vi "neuKLEIN.vi"() -> ()   [LabVIEW 2016] (continued)
"DIO2", "DIO3", "DIO4", "DIO5", "DIO6", "DIO7", "DIO8", "DIO9", "DIO10", "DIO11", "DIO12", "DIO13", "DIO14", "DIO15", "DIO16", "DIO17", "DIO18", "DIO19", "DIO20", "DIO21", "DIO22", "DIO23", "DIO24", "DIO25", "DIO26", "DIO27", "DIO28", "DIO29", "DIO30", "DIO31", "FALSE"]; "Channel 10"."Inputs" items=["DIO0", "DIO1", "DIO2", "DIO3", "DIO4", "DIO5", "DIO6", "DIO7", "DIO8", "DIO9", "DIO10", "DIO11", "DIO12", "DIO13", "DIO14", "DIO15", "DIO16", "DIO17", "DIO18", "DIO19", "DIO20", "DIO21", "DIO22", "DIO23", "DIO24", "DIO25", "DIO26", "DIO27", "DIO28", "DIO29", "DIO30", "DIO31", "FALSE"]; "Channel 10"."Operation" items=["OFF", "Constant", "Bool - Basic Switch", "Bool - AND Switch", "Bool - OR Switch", "Custom - Comp Basic Switch", "Custom - 461nm Freq."]; "Channel 9"."Input B" items=["DIO0", "DIO1", "DIO2", "DIO3", "DIO4", "DIO5", "DIO6", "DIO7", "DIO8", "DIO9", "DIO10", "DIO11", "DIO12", "DIO13", "DIO14", "DIO15", "DIO16", "DIO17", "DIO18", "DIO19", "DIO20", "DIO21", "DIO22", "DIO23", "DIO24", "DIO25", "DIO26", "DIO27", "DIO28", "DIO29", "DIO30", "DIO31", "FALSE"]; "Channel 9"."Input A" items=["DIO0", "DIO1", "DIO2", "DIO3", "DIO4", "DIO5", "DIO6", "DIO7", "DIO8", "DIO9", "DIO10", "DIO11", "DIO12", "DIO13", "DIO14", "DIO15", "DIO16", "DIO17", "DIO18", "DIO19", "DIO20", "DIO21", "DIO22", "DIO23", "DIO24", "DIO25", "DIO26", "DIO27", "DIO28", "DIO29", "DIO30", "DIO31", "FALSE"]; "Channel 9"."Inputs" items=["DIO0", "DIO1", "DIO2", "DIO3", "DIO4", "DIO5", "DIO6", "DIO7", "DIO8", "DIO9", "DIO10", "DIO11", "DIO12", "DIO13", "DIO14", "DIO15", "DIO16", "DIO17", "DIO18", "DIO19", "DIO20", "DIO21", "DIO22", "DIO23", "DIO24", "DIO25", "DIO26", "DIO27", "DIO28", "DIO29", "DIO30", "DIO31", "FALSE"]; "Channel 9"."Operation" items=["OFF", "Constant", "Bool - Basic Switch", "Bool - AND Switch", "Bool - OR Switch", "Custom - Comp Basic Switch", "Custom - 461nm Freq."]; "Channel 8"."Input B" items=["DIO0", "DIO1", "DIO2", "DIO3", "DIO4", "DIO5", "DIO6", "DIO7", "DIO8", "DIO9", "DIO10", "DIO11", "DIO12", "DIO13", "DIO14", "DIO15", "DIO16", "DIO17", "DIO18", "DIO19", "DIO20", "DIO21", "DIO22", "DIO23", "DIO24", "DIO25", "DIO26", "DIO27", "DIO28", "DIO29", "DIO30", "DIO31", "FALSE"]; "Channel 8"."Input A" items=["DIO0", "DIO1", "DIO2", "DIO3", "DIO4", "DIO5", "DIO6", "DIO7", "DIO8", "DIO9", "DIO10", "DIO11", "DIO12", "DIO13", "DIO14", "DIO15", "DIO16", "DIO17", "DIO18", "DIO19", "DIO20", "DIO21", "DIO22", "DIO23", "DIO24", "DIO25", "DIO26", "DIO27", "DIO28", "DIO29", "DIO30", "DIO31", "FALSE"]; "Channel 8"."Inputs" items=["DIO0", "DIO1", "DIO2", "DIO3", "DIO4", "DIO5", "DIO6", "DIO7", "DIO8", "DIO9", "DIO10", "DIO11", "DIO12", "DIO13", "DIO14", "DIO15", "DIO16", "DIO17", "DIO18", "DIO19", "DIO20", "DIO21", "DIO22", "DIO23", "DIO24", "DIO25", "DIO26", "DIO27", "DIO28", "DIO29", "DIO30", "DIO31", "FALSE"]; "Channel 8"."Operation" items=["OFF", "Constant", "Bool - Basic Switch", "Bool - AND Switch", "Bool - OR Switch", "Custom - Comp Basic Switch", "Custom - 461nm Freq."]; "Channel 7"."Input B" items=["DIO0", "DIO1", "DIO2", "DIO3", "DIO4", "DIO5", "DIO6", "DIO7", "DIO8", "DIO9", "DIO10", "DIO11", "DIO12", "DIO13", "DIO14", "DIO15", "DIO16", "DIO17", "DIO18", "DIO19", "DIO20", "DIO21", "DIO22", "DIO23", "DIO24", "DIO25", "DIO26", "DIO27", "DIO28", "DIO29", "DIO30", "DIO31", "FALSE"]; "Channel 7"."Input A" items=["DIO0", "DIO1", "DIO2", "DIO3", "DIO4", "DIO5", "DIO6", "DIO7", "DIO8", "DIO9", "DIO10", "DIO11", "DIO12", "DIO13", "DIO14", "DIO15", "DIO16", "DIO17", "DIO18", "DIO19", "DIO20", "DIO21", "DIO22", "DIO23", "DIO24", "DIO25", "DIO26", "DIO27", "DIO28", "DIO29", "DIO30", "DIO31", "FALSE"]; "Channel 7"."Inputs" items=["DIO0", "DIO1", "DIO2", "DIO3", "DIO4", "DIO5", "DIO6", "DIO7", "DIO8", "DIO9", "DIO10", "DIO11", "DIO12", "DIO13", "DIO14", "DIO15", "DIO16", "DIO17", "DIO18", "DIO19", "DIO20", "DIO21", "DIO22", "DIO23", "DIO24", "DIO25", "DIO26", "DIO27", "DIO28", "DIO29", "DIO30", "DIO31", "FALSE"]; "Channel 7"."Operation" items=["OFF", "Constant", "Bool - Basic Switch", "Bool - AND Switch", "Bool - OR Switch", "Custom - Comp Basic Switch", "Custom - 461nm Freq."]; "Channel 6"."Input B" items=["DIO0", "DIO1", "DIO2", "DIO3", "DIO4", "DIO5", "DIO6", "DIO7", "DIO8", "DIO9", "DIO10", "DIO11", "DIO12", "DIO13", "DIO14", "DIO15", "DIO16", "DIO17", "DIO18", "DIO19", "DIO20", "DIO21", "DIO22", "DIO23", "DIO24", "DIO25", "DIO26", "DIO27", "DIO28", "DIO29", "DIO30", "DIO31", "FALSE"]; "Channel 6"."Input A" items=["DIO0", "DIO1", "DIO2", "DIO3", "DIO4", "DIO5", "DIO6", "DIO7", "DIO8", "DIO9", "DIO10", "DIO11", "DIO12", "DIO13", "DIO14", "DIO15", "DIO16", "DIO17", "DIO18", "DIO19", "DIO20", "DIO21", "DIO22", "DIO23", "DIO24", "DIO25", "DIO26", "DIO27", "DIO28", "DIO29", "DIO30", "DIO31", "FALSE"]; "Channel 6"."Inputs" items=["DIO0", "DIO1", "DIO2", "DIO3", "DIO4", "DIO5", "DIO6", "DIO7", "DIO8", "DIO9", "DIO10", "DIO11", "DIO12", "DIO13", "DIO14", "DIO15", "DIO16", "DIO17", "DIO18", "DIO19", "DIO20", "DIO21", "DIO22", "DIO23", "DIO24", "DIO25", "DIO26", "DIO27", "DIO28", "DIO29", "DIO30", "DIO31", "FALSE"]; "Channel 6"."Operation" items=["OFF", "Constant", "Bool - Basic Switch", "Bool - AND Switch", "Bool - OR Switch", "Custom - Comp Basic Switch", "Custom - 461nm Freq."]; "Channel 5"."Input B" items=["DIO0", "DIO1", "DIO2", "DIO3", "DIO4", "DIO5", "DIO6", "DIO7", "DIO8", "DIO9", "DIO10", "DIO11", "DIO12", "DIO13", "DIO14", "DIO15", "DIO16", "DIO17", "DIO18", "DIO19", "DIO20", "DIO21", "DIO22", "DIO23", "DIO24", "DIO25", "DIO26", "DIO27", "DIO28", "DIO29", "DIO30", "DIO31", "FALSE"]; "Channel 5"."Input A" items=["DIO0", "DIO1", "DIO2", "DIO3", "DIO4", "DIO5", "DIO6", "DIO7", "DIO8", "DIO9", "DIO10", "DIO11", "DIO12", "DIO13", "DIO14", "DIO15", "DIO16", "DIO17", "DIO18", "DIO19", "DIO20", "DIO21", "DIO22", "DIO23", "DIO24", "DIO25", "DIO26", "DIO27", "DIO28", "DIO29", "DIO30", "DIO31", "FALSE"]; "Channel 5"."Inputs" items=["DIO0", "DIO1", "DIO2", "DIO3", "DIO4", "DIO5", "DIO6", "DIO7", "DIO8", "DIO9", "DIO10", "DIO11", "DIO12", "DIO13", "DIO14", "DIO15", "DIO16", "DIO17", "DIO18", "DIO19", "DIO20", "DIO21", "DIO22", "DIO23", "DIO24", "DIO25", "DIO26", "DIO27", "DIO28", "DIO29", "DIO30", "DIO31", "FALSE"]; "Channel 5"."Operation" items=["OFF", "Constant", "Bool - Basic Switch", "Bool - AND Switch", "Bool - OR Switch", "Custom - Comp Basic Switch", "Custom - 461nm Freq."]; "Channel 4"."Input B" items=["DIO0", "DIO1", "DIO2", "DIO3", "DIO4", "DIO5", "DIO6", "DIO7", "DIO8", "DIO9", "DIO10", "DIO11", "DIO12", "DIO13", "DIO14", "DIO15", "DIO16", "DIO17", "DIO18", "DIO19", "DIO20", "DIO21", "DIO22", "DIO23", "DIO24", "DIO25", "DIO26", "DIO27", "DIO28", "DIO29", "DIO30", "DIO31", "FALSE"]; "Channel 4"."Input A" items=["DIO0", "DIO1", "DIO2", "DIO3", "DIO4", "DIO5", "DIO6", "DIO7", "DIO8", "DIO9", "DIO10", "DIO11", "DIO12", "DIO13", "DIO14", "DIO15", "DIO16", "DIO17", "DIO18", "DIO19", "DIO20", "DIO21", "DIO22", "DIO23", "DIO24", "DIO25", "DIO26", "DIO27", "DIO28", "DIO29", "DIO30", "DIO31", "FALSE"]; "Channel 4"."Inputs" items=["DIO0", "DIO1", "DIO2", "DIO3", "DIO4", "DIO5", "DIO6", "DIO7", "DIO8", "DIO9", "DIO10", "DIO11", "DIO12", "DIO13", "DIO14", "DIO15", "DIO16", "DIO17", "DIO18", "DIO19", "DIO20", "DIO21", "DIO22", "DIO23", "DIO24", "DIO25", "DIO26", "DIO27", "DIO28", "DIO29", "DIO30", "DIO31", "FALSE"]; "Channel 4"."Operation" items=["OFF", "Constant", "Bool - Basic Switch", "Bool - AND Switch", "Bool - OR Switch", "Custom - Comp Basic Switch", "Custom - 461nm Freq."]; "Channel 3"."Input B" items=["DIO0", "DIO1", "DIO2", "DIO3", "DIO4", "DIO5", "DIO6", "DIO7", "DIO8", "DIO9", "DIO10", "DIO11", "DIO12", "DIO13", "DIO14", "DIO15", "DIO16", "DIO17", "DIO18", "DIO19", "DIO20", "DIO21", "DIO22", "DIO23", "DIO24", "DIO25", "DIO26", "DIO27", "DIO28", "DIO29", "DIO30", "DIO31", "FALSE"]; "Channel 3"."Input A" items=["DIO0", "DIO1", "DIO2", "DIO3", "DIO4", "DIO5", "DIO6", "DIO7", "DIO8", "DIO9", "DIO10", "DIO11", "DIO12", "DIO13", "DIO14", "DIO15", "DIO16", "DIO17", "DIO18", "DIO19", "DIO20", "DIO21", "DIO22", "DIO23", "DIO24", "DIO25", "DIO26", "DIO27", "DIO28", "DIO29", "DIO30", "DIO31", "FALSE"]; "Channel 3"."Inputs" items=["DIO0", "DIO1", "DIO2", "DIO3", "DIO4", "DIO5", "DIO6", "DIO7", "DIO8", "DIO9", "DIO10", "DIO11", "DIO12", "DIO13", "DIO14", "DIO15", "DIO16", "DIO17", "DIO18", "DIO19", "DIO20", "DIO21", "DIO22", "DIO23", "DIO24", "DIO25", "DIO26", "DIO27", "DIO28", "DIO29", "DIO30", "DIO31", "FALSE"]; "Channel 3"."Operation" items=["OFF", "Constant", "Bool - Basic Switch", "Bool - AND Switch", "Bool - OR Switch", "Custom - Comp Basic Switch", "Custom - 461nm Freq."]; "Channel 2"."Input B" items=["DIO0", "DIO1", "DIO2", "DIO3", "DIO4", "DIO5", "DIO6", "DIO7", "DIO8", "DIO9", "DIO10", "DIO11", "DIO12", "DIO13", "DIO14", "DIO15", "DIO16", "DIO17", "DIO18", "DIO19", "DIO20", "DIO21", "DIO22", "DIO23", "DIO24", "DIO25", "DIO26", "DIO27", "DIO28", "DIO29", "DIO30", "DIO31", "FALSE"]; "Channel 2"."Input A" items=["DIO0", "DIO1", "DIO2", "DIO3", "DIO4", "DIO5", "DIO6", "DIO7", "DIO8", "DIO9", "DIO10", "DIO11", "DIO12", "DIO13", "DIO14", "DIO15", "DIO16", "DIO17", "DIO18", "DIO19", "DIO20", "DIO21", "DIO22", "DIO23", "DIO24", "DIO25", "DIO26", "DIO27", "DIO28", "DIO29", "DIO30", "DIO31", "FALSE"]; "Channel 2"."Inputs" items=["DIO0", "DIO1", "DIO2", "DIO3", "DIO4", "DIO5", "DIO6", "DIO7", "DIO8", "DIO9", "DIO10", "DIO11", "DIO12", "DIO13", "DIO14", "DIO15", "DIO16", "DIO17", "DIO18", "DIO19", "DIO20", "DIO21", "DIO22", "DIO23", "DIO24", "DIO25", "DIO26", "DIO27", "DIO28", "DIO29", "DIO30", "DIO31", "FALSE"]; "Channel 2"."Operation" items=["OFF", "Constant", "Bool - Basic Switch", "Bool - AND Switch", "Bool - OR Switch", "Custom - Comp Basic Switch", "Custom - 461nm Freq."]; "Channel 1"."Input B" items=["DIO0", "DIO1", "DIO2", "DIO3", "DIO4", "DIO5", "DIO6", "DIO7", "DIO8", "DIO9", "DIO10", "DIO11", "DIO12", "DIO13", "DIO14", "DIO15", "DIO16", "DIO17", "DIO18", "DIO19", "DIO20", "DIO21", "DIO22", "DIO23", "DIO24", "DIO25", "DIO26", "DIO27", "DIO28", "DIO29", "DIO30", "DIO31", "FALSE"]; "Channel 1"."Input A" items=["DIO0", "DIO1", "DIO2", "DIO3", "DIO4", "DIO5", "DIO6", "DIO7", "DIO8", "DIO9", "DIO10", "DIO11", "DIO12", "DIO13", "DIO14", "DIO15", "DIO16", "DIO17", "DIO18", "DIO19", "DIO20", "DIO21", "DIO22", "DIO23", "DIO24", "DIO25", "DIO26", "DIO27", "DIO28", "DIO29", "DIO30", "DIO31", "FALSE"]; "Channel 1"."Inputs" items=["DIO0", "DIO1", "DIO2", "DIO3", "DIO4", "DIO5", "DIO6", "DIO7", "DIO8", "DIO9", "DIO10", "DIO11", "DIO12", "DIO13", "DIO14", "DIO15", "DIO16", "DIO17", "DIO18", "DIO19", "DIO20", "DIO21", "DIO22", "DIO23", "DIO24", "DIO25", "DIO26", "DIO27", "DIO28", "DIO29", "DIO30", "DIO31", "FALSE"]; "Channel 1"."Operation" items=["OFF", "Constant", "Bool - Basic Switch", "Bool - AND Switch", "Bool - OR Switch", "Custom - Comp Basic Switch", "Custom - 461nm Freq."]; "Channel 0"."Input B" items=["DIO0", "DIO1", "DIO2", "DIO3", "DIO4", "DIO5", "DIO6", "DIO7", "DIO8", "DIO9", "DIO10", "DIO11", "DIO12", "DIO13", "DIO14", "DIO15", "DIO16", "DIO17", "DIO18", "DIO19", "DIO20", "DIO21", "DIO22", "DIO23", "DIO24", "DIO25", "DIO26", "DIO27", "DIO28", "DIO29", "DIO30", "DIO31", "FALSE"]; "Channel 0"."Input A" items=["DIO0", "DIO1", "DIO2", "DIO3", "DIO4", "DIO5", "DIO6", "DIO7", "DIO8", "DIO9", "DIO10", "DIO11", "DIO12", "DIO13", "DIO14", "DIO15", "DIO16", "DIO17", "DIO18", "DIO19", "DIO20", "DIO21", "DIO22", "DIO23", "DIO24", "DIO25", "DIO26", "DIO27", "DIO28", "DIO29", "DIO30", "DIO31", "FALSE"]; "Channel 0"."Inputs" items=["DIO0", "DIO1", "DIO2", "DIO3", "DIO4", "DIO5", "DIO6", "DIO7", "DIO8", "DIO9", "DIO10", "DIO11", "DIO12", "DIO13", "DIO14", "DIO15", "DIO16", "DIO17", "DIO18", "DIO19", "DIO20", "DIO21", "DIO22", "DIO23", "DIO24", "DIO25", "DIO26", "DIO27", "DIO28", "DIO29", "DIO30", "DIO31", "FALSE"]; "Channel 0"."Operation" items=["OFF", "Constant", "Bool - Basic Switch", "Bool - AND Switch", "Bool - OR Switch", "Custom - Comp Basic Switch", "Custom - 461nm Freq."]}
  in  "FPGA_Labels":T34={"Channel 0"={"Channel Description"="This channel is outputtnig a constant voltage for unknown reasons\n- Jim\n2018.04.24"}, "Channel 1"={"Channel Description"="This channel is outputtnig a constant voltage for unknown reasons\n- Jim\n2018.04.24"}, "Channel 2"={"Channel Description"="Blue MOT Field Gradient"}, "Channel 3"={"Channel Description"="6221 Waveform trigger\n\nODT card that is triggered if either the sheet or the loading trap is turned on"}, "Channel 4"={"Channel Description"="X Trim Coil\nUsing Bio chip supply\n\n2018.04.12 - Zero field value\n-0.109985 V\n"}, "Channel 6"={"Channel Description"="Z Trim Coil\nUsing Gwinstek 5A supply\n\n2018.04.12 - Zero field value\n1.21 V\n\nODT loading value - 1.175 V\n2018.07.12 - Trapping 87\nTrap final: 81.8 MHz\nStir final:  143.605 MHz"}, "Channel 5"={"Channel Description"="Y Trim Coil\nUsing Gwinstek 3A supply\n\n2018.04.12 - Zero field value\n1.5 V\n"}, "Channel 7"={"Channel Description"="LCR Control\n\nDefining a coord systme with +Bz anti-parallel to gravity then\n\nSigma Plus:      1.75V\nSigma Minus:   0.95V"}, "Channel 8"={"Channel Description"="Blue Laser Frequency Selector\n\nSingle isotope without Cold MOT frequency shift can use the Bool - Basic switch operation\n\nDual isotopr or use of the Cold MOT freq shift should use the Custom 461nm Freq operation\n\nBool - Basic Switch op Outputs\nHI - Trap Freq.\nLO - Image Freq.\n\nCustom op Outputs:\n0 - Image Freq. 0\n1 - Image Freq. 1\n2 - Cold MOT Trap Freq\n3 - Hot MOT Trap Freq 0\n4 - Hot MOT Trap Freq 1\n"}, "Channel 9"={"Channel Description"="Blue MOT Power Control"}, "Channel 10"={"Channel Description"=""}, "Channel 11"={"Channel Description"=""}, "Channel 12"={"Channel Description"=""}, "Channel 13"={"Channel Description"=""}, "Channel 14"={"Channel Description"=""}, "Channel 15"={"Channel Description"=""}}
  in  "Synth Notes":string="- When scanning\nPhase to Change picks which synth to vary\nChannel to change picks the synth channel\n--------------------------------------------------------------------------\nNOTE: Signs below indicate the orientation of the AOM\n689 Master is locked -82 MHz of the 88Sr transition\n--------------------------------------------------------------------------\n## Constant values (i.e. important and generally unchanging)\n## Old sat abs parameters\n- Red Sat Abs. Freqs, Chan0: -81.85 MHz, Chan1: -82.15 MHz\n\n## New sat abs synth params as of 2018.08.22\n- Red Sat Abs. Chan0: 81.5MHz 1Vpp, Chan1: 82.5MHz 0.75Vpp\n\n- Isotope Selector AOM Freqs (2017.10.02)\n(note this value is sent through a doubler before gonig to the AOM)\n84Sr:  -93.745 MHz (\n86Sr:  no shift\n88Sr:  +82 MHz\n\n- Red MOT Single Freq. Resonances (2018.05.14)\nBoson: -82 MHz\nTrap: +82 MHz\nStir: +143.71 MHz\n\n- Slave 1 Inj. Freq  (2018.07.12),  +160 MHz \n\n--------------------------------------------------------------------------\n## Experimental Setting notes\n"
  in  "Novatech Synth Settings":T36[][](array[typedef])=[[{"Channel Settings"=[{"Voltage (Amp.) "=0.1, "Frequency (MHz)"=143.6, "Phase (deg)"=0.0, "Nickname"="SpinPol HI-Pump"}, {"Voltage (Amp.) "=1.0, "Frequency (MHz)"=0.0, "Phase (deg)"=0.0, "Nickname"="reserved for TM"}, {"Voltage (Amp.) "=0.1, "Frequency (MHz)"=145.0, "Phase (deg)"=0.0, "Nickname"="SpinPol LO-Probe"}, {"Voltage (Amp.) "=1.0, "Frequency (MHz)"=40.0, "Phase (deg)"=0.0, "Nickname"="Spec Offset Freq."}], "Active Chans"=[FALSE, FALSE, FALSE, TRUE], "COM Port"="ntSynth_COM5", "Table Mode"={"Initial Freq.(MHz)"=142.4, "FinalFreq"=145.32, "Freq. Step (MHz)"=0.365, "Voltage (Amp.)"=0.1, "Asc. & Desc."=FALSE, "Custom Frequencies"=[], "Custom Amplitude"=[], "Table Mode Switch"=FALSE, "Array Gen"=enum."Auto", "Randomize"=FALSE, "Continuous"=FALSE}}, {"Channel Settings"=[{"Voltage (Amp.) "=1.0, "Frequency (MHz)"=81.5, "Phase (deg)"=0.0, "Nickname"="Red Sat Abs - Chan0"}, {"Voltage (Amp.) "=0.97, "Frequency (MHz)"=82.5, "Phase (deg)"=0.0, "Nickname"="Red Sat Abs - Chan1"}, {"Voltage (Amp.) "=0.0, "Frequency (MHz)"=93.745, "Phase (deg)"=0.0, "Nickname"="Isotope Sel. AOM"}, {"Voltage (Amp.) "=0.28, "Frequency (MHz)"=160.0, "Phase (deg)"=0.0, "Nickname"="Slave 1 Inj. Freq"}], "Active Chans"=[FALSE, FALSE, FALSE, FALSE], "COM Port"="ntSynth_COM6", "Table Mode"={"Initial Freq.(MHz)"=0.0, "FinalFreq"=0.0, "Freq. Step (MHz)"=0.0, "Voltage (Amp.)"=0.0, "Asc. & Desc."=FALSE, "Custom Frequencies"=[], "Custom Amplitude"=[], "Table Mode Switch"=FALSE, "Array Gen"=enum."Auto", "Randomize"=FALSE, "Continuous"=FALSE}}], [{"Channel Settings"=[{"Voltage (Amp.) "=1.0, "Frequency (MHz)"=82.015, "Phase (deg)"=0.0, "Nickname"="Red Boson SF"}, {"Voltage (Amp.) "=1.0, "Frequency (MHz)"=100.0, "Phase (deg)"=0.0, "Nickname"="BROKEN"}, {"Voltage (Amp.) "=1.0, "Frequency (MHz)"=81.93, "Phase (deg)"=0.0, "Nickname"="Red 87 SF Trap"}, {"Voltage (Amp.) "=1.0, "Frequency (MHz)"=143.715, "Phase (deg)"=0.0, "Nickname"="Red 87 SF Stir"}], "Active Chans"=[TRUE, FALSE, TRUE, TRUE], "COM Port"="ntSynth_COM11", "Table Mode"={"Initial Freq.(MHz)"=0.17, "FinalFreq"=81.95, "Freq. Step (MHz)"=0.175, "Voltage (Amp.)"=0.0, "Asc. & Desc."=FALSE, "Custom Frequencies"=[], "Custom Amplitude"=[], "Table Mode Switch"=FALSE, "Array Gen"=enum."Auto", "Randomize"=FALSE, "Continuous"=FALSE}}, {"Channel Settings"=[{"Voltage (Amp.) "=0.22, "Frequency (MHz)"=85.95, "Phase (deg)"=0.0, "Nickname"="Spec. 1 Freq 0 (LO)"}, {"Voltage (Amp.) "=0.22, "Frequency (MHz)"=85.85, "Phase (deg)"=0.0, "Nickname"="Spec. 1 Freq 1 (HI)"}, {"Voltage (Amp.) "=1.0, "Frequency (MHz)"=93.745, "Phase (deg)"=0.0, "Nickname"="Bragg - 1"}, {"Voltage (Amp.) "=1.0, "Frequency (MHz)"=90.0, "Phase (deg)"=0.0, "Nickname"="Bragg - 2"}], "Active Chans"=[TRUE, TRUE, FALSE, FALSE], "COM Port"="ntSynth_COM10", "Table Mode"={"Initial Freq.(MHz)"=81.95, "FinalFreq"=82.05, "Freq. Step (MHz)"=0.002, "Voltage (Amp.)"=1.0, "Asc. & Desc."=TRUE, "Custom Frequencies"=[], "Custom Amplitude"=[], "Table Mode Switch"=FALSE, "Array Gen"=enum."Auto", "Randomize"=FALSE, "Continuous"=TRUE}}]] {"Table Mode"."Freq. Step (MHz)" format="%#_9g"; "Table Mode"."FinalFreq" format="%#_9g"; "Table Mode"."Initial Freq.(MHz)" format="%#_9g"; "Channel Settings"."Frequency (MHz)" format="%#_9g"}
  in  "Intitialize PicoScope":bool
  in  "PicoScope":T39={"Channel A Settings"={"Enabled"=FALSE, "Coupling"=1, "Range"=6, "Analogue Offset"=0.0}, "Channel B Settings"={"Enabled"=TRUE, "Coupling"=1, "Range"=8, "Analogue Offset"=0.0}, "Trigger Options"={"Trigger Enabled"=TRUE, "Trigger Source"=enum."Ext.", "Trigger Threshold (-5 to 5 V)"=1.0, "Trigger Slope"=2, "Trigger Delay (s)"=0.0, "Auto Trigger Time (ms)"=5000}, "Pico Scope Inititalization Settings"={"USB Power"=TRUE, "Use Serial Number"=FALSE, "Resolution"=3, "Serial Number"="", "Handle"=16384}, "Use PicoScope?"=FALSE, "Acquisition Settings"={"Pre Trigger Time (s)"=0.0, "Post Trigger Time (s)"=0.2, "Resolution (s)"=1e-06, "Four Channel Device"=FALSE, "Number of Captures"=1.0}} {"Acquisition Settings"."Number of Captures" min=1.0 step=1.0; "Acquisition Settings"."Resolution (s)" min=8e-09 max=34.36 step=8e-09 format="%#_6p"; "Acquisition Settings"."Post Trigger Time (s)" min=0.0 format="%#_6p"; "Acquisition Settings"."Pre Trigger Time (s)" min=0.0 format="%#_6p"; "Pico Scope Inititalization Settings"."Resolution" items=["8-bit", "12-bit", "14-bit", "15-bit (max. 2 ch.)", "16-bit (max. 1 ch.)"]; "Trigger Options"."Trigger Delay (s)" format="%.0p"; "Trigger Options"."Trigger Slope" items=["Rising"=2, "Falling"=3]; "Trigger Options"."Trigger Threshold (-5 to 5 V)" format="%.2f"; "Channel B Settings"."Range" items=["10 mV", "20 mV", "50 mV", "100 mV", "200 mV", "500 mV", "1 V", "2 V", "5 V", "10 V", "20 V", "50 V ", "100 V"]; "Channel B Settings"."Coupling" items=["AC", "DC"]; "Channel A Settings"."Range" items=["10 mV", "20 mV", "50 mV", "100 mV", "200 mV", "500 mV", "1 V", "2 V", "5 V", "10 V", "20 V", "50 V ", "100 V"]; "Channel A Settings"."Coupling" items=["AC", "DC"]}
  in  "Program Agilent":bool
  in  "Agilent E3631A Settings":T43={"VISA resource name"="Agilent_Trim_Supply", "Voltage Set (6V max)"=6.0, "Current Set (5A max)"=0.013, "Voltage Set (25V max)"=25.0, "Current Set (1A max)"=0.273, "Voltage Set (-25V max)"=-25.0, "Current Set (1A max)"=0.555, "6V Switch"=TRUE, "+25V Switch"=TRUE, "-25V Switch"=FALSE, "Agilent E3631A Measurements"={"6V Actual Voltage Level (V)"=0.02291032, "6V Actual Current Level (A)"=0.01098386, "25V Actual Voltage Level (V)"=0.4245154, "25V Actual Current Level (A)"=0.2743926, "-25V Actual Current Level (A)"=0.0, "-25V Actual Voltage Level (V)"=0.0}, "Triggered Agilent Settings"={"Trigger \nDelay (s)"=3.0, "Enable +6V Channel"=TRUE, "+6V Current"=0.02, "Enable -25V Channel"=TRUE, "-25V Current"=0.0, "Enable +25V Channel"=TRUE, "+25V Current"=0.275}, "Auto Program Agilent"=FALSE, "Agilent Software Trigger"=FALSE} {"Triggered Agilent Settings"."Trigger \nDelay (s)" min=0.0 max=3600.0 step=1.0 format="%.2f"; "Agilent E3631A Measurements"."-25V Actual Current Level (A)" format="%.3g"; "Agilent E3631A Measurements"."-25V Actual Voltage Level (V)" format="%.3g"; "Agilent E3631A Measurements"."25V Actual Current Level (A)" format="%.3g"; "Agilent E3631A Measurements"."25V Actual Voltage Level (V)" format="%.3g"; "Agilent E3631A Measurements"."6V Actual Current Level (A)" format="%.3g"; "Agilent E3631A Measurements"."6V Actual Voltage Level (V)" format="%.3g"; "Current Set (1A max)" format="%.3g"; "Voltage Set (-25V max)" format="%.3g"; "Current Set (1A max)" format="%.3g"; "Voltage Set (25V max)" format="%.3g"; "Current Set (5A max)" format="%.3g"; "Voltage Set (6V max)" format="%.3g"}
  in  "SaveButton":bool
  in  "XML Filename":string="20181207 - Settings 2"
  in  "Load":bool
  in  "XML File Location":path=path "Z:/Neutral/Experiment_Data/NeuKLEIN XML Configs/20181206 - test3 - SpinalCol MD5 0d3911740401e8bd5a903395efd23ac1.dat"
  out "current spinal_column MD5":string="0d3911740401e8bd5a903395efd23ac1"
  out "cRIO Ready":bool
  out "Picoscope Ready":bool
  in  "Break Loop":bool
  in  "Abort Scan":bool
  in  "Take Pictures":bool=TRUE
  in  "Trigger Snap Mode":bool=TRUE
  in  "Shutdown Experiment":bool
  in  "Start Experiment":bool
  out "Camera Ready":bool=TRUE
  out "Exp Running":bool
  in  "output cluster":T46
  in  "Stats Flag":bool
  out "Num and Temp Stats":T47 {"Std. Y Temp" format="%#_3p"; "Mean Y Temp" format="%#_3p"; "Mean X Temp" format="%#_3p"; "Mean Num." format="%^#.3e"; "Std. X Temp" format="%#_3p"; "Std. Num" format="%^#.3e"}
  in  "Stat. Limits":cluster{"Start Index":dbl, "Length":dbl}={"Start Index"=1738.0, "Length"=1000.0}
  out "Wavemeter":string="1"
  out "Phase Space Density":dbl=5.84831043500419e-05 format="%#_3e"
  in  "Trap Frequencies":T48={"w_x [Hz]"=27.6, "w_y [Hz]"=15.4, "w_z [Hz]"=219.0}
  out "Scan Name":string="87Sr_gODT_1P1PAS_Lifetime_load-10s_461Freq-21698.057cm-1_pdSet-8.5V_1631"
  out "Scan Progress":T49
  in  "Drop Time":dbl=0.012 min=1e-06 format="%#_6p"
  out "Temp. (K) - Y":dbl=2.294660734428253e-06 format="%#.2p"
  out "Temp. (K) - X":dbl=2.785132808461954e-06 format="%#.2p"
  in  "Set Analysis Mode":enum16{"Fast", "Fancy"}(ring)=enum."Fancy"
  out "Number":dbl=91830.26185483216 format="%^#.3g"
  out "Current Param. Values":dbl[](array[numeric]) format="%^#.3e"
  in  "Information Tab Control":T50(tab)
  out "Temperature Chart":T51(graph)={"Temperature (K) x"=2.785132808461954e-06, "Temperature (K) y"=2.294660734428253e-06} caption="Waveform Chart"
  out "Best Fit Parameter Cluster":T52={"Amplitude (OD)"=0.04212355745219539, "X Center (px)"=36.66813300766018, "Y Center (px)"=27.147499594349803, " X Width (um)"=196.94453372331347, "Y Width (um)"=178.76406377906994, "Aspect Ratio"=1.1017009210906745, "Rot. Angle (deg)"=14.77510547044796} {"Rot. Angle (deg)" format="%#.3g"; "Aspect Ratio" format="%#.3g"; "Y Width (um)" format="%#.3g"; "X Width (um)" format="%#.3g"; "Y Center (px)" format="%#.3g"; "X Center (px)" format="%#.3g"; "Amplitude (OD)" format="%#.3g"}
  out "Data Cuts":dbl[][](graph)=[[-0.018516517706997773, -0.018194611112609834, -0.017792111984277766, -0.0172946162259058, -0.016686833508987226, -0.015953029842122612, -0.01507761558608454, -0.014045878123250102, -0.01284484691296142, -0.011464265374227347, -0.00989762980768302, -0.008143241586180698, -0.0062052065371251686, -0.0040943063647016185, -0.0018286626382211027, 0.000565884394490665, 0.003055751235310024, 0.00559999395959896, 0.00815112886297439, 0.010656393022784885, 0.013059414875679881, 0.015302231843355198, 0.017327560865164682, 0.019081201496622048, 0.020514432848943213, 0.02158625734302467, 0.022265347425911908, 0.022531566360891882, 0.022376960092342038, 0.02180615201432442, 0.020836113303899118, 0.019495324738332355, 0.0178223877595797, 0.015864179292424896, 0.01367367332602995, 0.011307570269025746, 0.008823881414105308, 0.006279610502850457, 0.003728658487908019, 0.0012200532082126195, -0.0012034244550768597, -0.0035061792398605185, -0.005660298829146124, -0.007645633216064877, -0.009449503849510243, -0.011066108099310294, -0.012495695177412305, -0.01374359316453528, -0.014819163966026245, -0.01573475506633155, -0.016504705350745216, -0.017144448579056948, -0.017669743804466495, -0.018096048392369418, -0.01843803726813114, -0.01870926223753828, -0.01892193797824844, -0.019086836608532706, 0.0, 0.0, 0.0, 0.0, 0.0, 0.0, 0.0, 0.0, 0.0, 0.0], [-0.019427195823243468, -0.019376477281740065, -0.019309777651095317, -0.01922287093556023, -0.019110685721095158, -0.01896722020910829, -0.018785474537675276, -0.018557409904020224, -0.018273945208152165, -0.017925002694703936, -0.01749961417579863, -0.01698609867123254, -0.01637232052539525, -0.015646034123077857, -0.014795317173077124, -0.013809089203456868, -0.012677705579914374, -0.011393610315763865, -0.009952023618114425, -0.008351633057735204, -0.006595251095550987, -0.0046903971238530726, -0.0026497598438430803, -0.0004914962743148774, 0.0017606726186124855, 0.00407760257670621, 0.006425125473125102, 0.008764716644499147, 0.01105442371575498, 0.013250033718289263, 0.015306438490773934, 0.01717914283317453, 0.01882584698418749, 0.020208025915155796, 0.021292423639983432, 0.02205238183925677, 0.022468928766872162, 0.022531566360891882, 0.022238709969994795, 0.021597754981757165, 0.020624766441733944, 0.01934380984938667, 0.017785962047794715, 0.015988058953357864, 0.013991250527588636, 0.011839441977871928, 0.009577703234884861, 0.007250726308140266, 0.0049014026324586575, 0.0025695808347483383, 0.00029105060475955943, -0.0019032181567382456, -0.003987568677420049, -0.005941887018274791, -0.007751586238736624, -0.009407374627950797, -0.010904845904679735, -0.01224393417407418, -0.013428277998825504, -0.014464536535176719, -0.01536169682432155, -0.01613040565297022, -0.016782352581386856, -0.01732972343932546, -0.017784736393057377, -0.018159266063668068, -0.018464555472172003, -0.018711011010899024], [-0.019674183393878053, -0.018280247132970828, -0.03707034333922188, -0.011839983562165202, -0.016998709481589103, -0.012341104046555529, -0.021997574754431426, -0.009335227908014332, -0.022468248671767554, -0.008841936710549447, -0.004166380111126244, -0.0036079885407822587, 0.013868297756534531, 0.004561068478993846, 0.006293340497313338, -0.014363456038362088, 0.017193001345752634, 0.006093376204407974, -0.0024781042376211815, 0.011271825696079318, 0.008691889664444119, 0.011941615562930608, 0.023012521272605113, 0.0019642863458724236, 0.017272880112823685, 0.016136631094548548, 0.008687918506820935, 0.02099221280840169, 0.017917862798283224, 0.009631050809833397, 0.02554609242769601, 0.04013080877613362, 0.026291061942652405, 0.02539649470299743, 0.02706597230576513, 0.011647790022525584, 0.008213130067025176, 0.0008036375604341117, -0.0042861821776742914, -0.0025318843232824406, 0.0017634568314921495, -0.0005986557636141754, -0.0058368393092997906, 0.00508266964400228, -0.00835695832072858, -0.018218434170771403, -0.017155286275254866, -0.014485423881440695, -0.019467133583539464, -0.013682561116603154, -0.006443282460669053, -0.009833326613170712, -0.02184413355864656, -0.02296819550088358, -0.006375659160697822, -0.015850956409911632, -0.004489345362594932, -0.02235341217838993, 0.0, 0.0, 0.0, 0.0, 0.0, 0.0, 0.0, 0.0, 0.0, 0.0], [-0.0243737584562691, -0.017111035311295097, -0.022859847372362907, -0.010456022312313351, -0.018621764294113774, -0.010363258058342595, -0.01924017207365125, -0.005392739464966212, -0.001821858354572825, -0.013500239832344718, -0.02316427859648229, -0.023003857627395874, -0.019410330233691653, -0.02366483034358069, -0.020338383323426967, -0.012296466042950982, -0.00805826010824795, -0.0004434589873110184, -0.008477287816239354, -0.011745997299295041, -0.013598201777075047, -0.014398642561154418, 0.0015444972643692267, -0.0006483823089116214, 0.010682715509897633, 0.002583130060950012, -0.0009655052097361505, 0.008919591817919681, 0.023429159753034057, 0.011608219160690325, 0.021082652933930746, 0.03492013623202617, 0.03166850362650919, 0.02933973934800882, 0.028860413280865416, 0.016524774616293314, 0.027570668641088147, 0.02099221280840169, 0.004148948809319819, 0.020613558739894344, 0.027621676607532564, 0.01739174271186883, 0.006233170598839877, 0.007901766107952568, 0.025351591197415146, 0.009984160055523716, 0.0022128081997880855, 0.004184214591864688, -0.0016938681459777172, -0.006981538615955074, -0.018690254673993323, -0.00559181326577729, -0.001978729312451577, -0.006617235862030668, 0.0063716224206622485, 0.005566298593278063, -0.009026165183652068, -0.000989707127500239, 0.005242246944712647, -0.013162148630106785, -0.005795760157143448, -0.015456414382502004, -0.022333780847009876, -0.016806338004888843, -0.018674418764843992, -0.013384730813303491, 0.000991629561818641, -0.0011573756424354542]]
  out "Atoms - BG":dbl[][](graph)